vi "FlexMag - 24-03-2023.vi"() -> ()   [LabVIEW 2018] (continued)
                                }
                                frame True {
                                n21945 = Wait (ms)(milliseconds to wait=u32 100) -> ()  [unwired: 1 out]
                                "coating ch4 led 6" <- TRUE ("coating ch2 led 1")
                                }
                                }
                                }
                                frame True {
                                }
                                }
                                }
                                }
                                }
                                frame #7 {
                                # "baratron bv open"
                                n21946 = stacked-sequence {
                                frame #0 {
                                n21947 = local read "abort ch4"() -> (w25919:bool)
                                n21948 = case shown="False" w25919 {
                                frame False {
                                n21949 = local read "coating start"() -> (w25920:bool)
                                n21950 = case shown="True" w25920 {
                                frame False {
                                }
                                frame True {
                                n21951 = while {
                                i -> [w25923]
                                stop <- w25925 stop-if-true
                                n21952 = Greater Or Equal?(x=w25923, y=100) -> (x >= y?=w25924:bool)
                                n21953 = case shown="True" w25924 {
                                frame False {
                                }
                                frame True {
                                n21954 = local write "Warning Message"("Automatic Coating Process is canceled !\nCH4 Baratron Gauge Block Valve couldn't be opned.." ("Warning Message")) -> ()
                                n21955 = local write "coating error"(TRUE ("coating error")) -> ()
                                }
                                }
                                n21956 = local read "CH4_BG_BV_DI"() -> (w25929:bool)
                                n21957 = case shown="False" w25929 {
                                tunnel: [FALSE ("CH2_WFC_DO") TRUE ("CH2_WFC_DO")] -> w25928
                                frame False {
                                n21958 = Wait Until Next ms Multiple(millisecond multiple=u32 200) -> ()  [unwired: 1 out]
                                n21959 = local write "CH4_BG_BV_DO"(TRUE ("coating error")) -> ()
                                }
                                frame True {
                                }
                                }
                                n21960 = local read "coating start"() -> (w25927:bool)
                                n21961 = local read "abort ch4"() -> (w25921:bool)
                                n21962 = Not(x=w25927) -> (.not. x?=w25926:bool)
                                n21963 = Compound Arithmetic op=OR(w25928, w25926, w25921) -> (w25925:bool)
                                }
                                }
                                }
                                }
                                frame True {
                                }
                                }
                                }
                                frame #1 {
                                n21964 = local read "abort ch4"() -> (w25936:bool)
                                n21965 = case shown="False" w25936 {
                                frame False {
                                n21966 = local read "coating start"() -> (w25937:bool)
                                n21967 = case shown="True" w25937 {
                                frame False {
                                }
                                frame True {
                                n21968 = Wait (ms)(milliseconds to wait=u32 100) -> ()  [unwired: 1 out]
                                "coating ch4 led 7" <- TRUE ("coating ch2 led 1")
                                }
                                }
                                }
                                frame True {
                                }
                                }
                                }
                                }
                                }
                                frame #8 {
                                # "ar sov open"
                                n21969 = stacked-sequence {
                                frame #0 {
                                n21970 = local read "abort ch4"() -> (w25940:bool)
                                n21971 = case shown="False" w25940 {
                                frame False {
                                n21972 = local read "coating start"() -> (w25941:bool)
                                n21973 = case shown="True" w25941 {
                                frame False {
                                }
                                frame True {
                                n21974 = while {
                                i -> [w25944]
                                stop <- w25946 stop-if-true
                                n21975 = Greater Or Equal?(x=w25944, y=100) -> (x >= y?=w25945:bool)
                                n21976 = case shown="True" w25945 {
                                frame False {
                                }
                                frame True {
                                n21977 = local write "Warning Message"("Automatic Coating Process is canceled !\nCH4 SoV Ar couldn't be opened.." ("Warning Message")) -> ()
                                n21978 = local write "coating error"(TRUE ("coating error")) -> ()
                                }
                                }
                                n21979 = local read "CH4_SoV_Ar_DI"() -> (w25950:bool)
                                n21980 = case shown="False" w25950 {
                                tunnel: [FALSE ("CH2_WFC_DO") TRUE ("CH2_WFC_DO")] -> w25949
                                frame False {
                                n21981 = Wait Until Next ms Multiple(millisecond multiple=u32 200) -> ()  [unwired: 1 out]
                                n21982 = local write "CH4_SoV_Ar_DO"(TRUE ("coating error")) -> ()
                                }
                                frame True {
                                }
                                }
                                n21983 = local read "coating start"() -> (w25948:bool)
                                n21984 = local read "abort ch4"() -> (w25942:bool)
                                n21985 = Not(x=w25948) -> (.not. x?=w25947:bool)
                                n21986 = Compound Arithmetic op=OR(w25949, w25947, w25942) -> (w25946:bool)
                                }
                                }
                                }
                                }
                                frame True {
                                }
                                }
                                }
                                frame #1 {
                                n21987 = local read "abort ch4"() -> (w25957:bool)
                                n21988 = case shown="False" w25957 {
                                frame False {
                                n21989 = local read "coating start"() -> (w25958:bool)
                                n21990 = case shown="True" w25958 {
                                frame False {
                                }
                                frame True {
                                n21991 = Wait (ms)(milliseconds to wait=u32 100) -> ()  [unwired: 1 out]
                                "coating ch4 led 8" <- TRUE ("coating ch2 led 1")
                                }
                                }
                                }
                                frame True {
                                }
                                }
                                }
                                }
                                }
                                frame #9 {
                                # "mfc set"
                                n21992 = stacked-sequence {
                                frame #0 {
                                n21993 = local read "abort ch4"() -> (w25961:bool)
                                n21994 = case shown="False" w25961 {
                                frame False {
                                n21995 = local read "coating start"() -> (w25962:bool)
                                n21996 = case shown="True" w25962 {
                                frame False {
                                }
                                frame True {
                                n21997 = flat-sequence {
                                frame #0 {
                                n21998 = local read "R Ar set sccm"() -> (w25964:dbl)
                                n21999 = local write "ch4 argon mfc set"(w25964) -> ()
                                n22000 = Wait (ms)(milliseconds to wait=u32 300) -> ()  [unwired: 1 out]
                                }
                                frame #1 {
                                n22001 = local write "ch4 ar set auto"(TRUE ("ch2 ar set auto")) -> ()
                                }
                                }
                                }
                                }
                                }
                                frame True {
                                }
                                }
                                }
                                frame #1 {
                                n22002 = local read "abort ch4"() -> (w25966:bool)
                                n22003 = case shown="False" w25966 {
                                frame False {
                                n22004 = local read "coating start"() -> (w25967:bool)
                                n22005 = case shown="True" w25967 {
                                frame False {
                                }
                                frame True {
                                n22006 = while {
                                i -> [w25977]
                                stop <- w25979 stop-if-true
                                n22007 = local read "R Ar set sccm"() -> (w25973:dbl)
                                n22008 = Greater Or Equal?(x=w25977, y=50) -> (x >= y?=w25978:bool)
                                n22009 = case shown="True" w25978 {
                                frame False {
                                }
                                frame True {
                                n22010 = local write "Warning Message"("Automatic Coating Process is canceled !\nCH4  MFC Ar flow problem..." ("Warning Message")) -> ()
                                n22011 = local write "coating error"(TRUE ("coating error")) -> ()
                                }
                                }
                                n22012 = local read "ch4 argon mfc actual"() -> (w25974:dbl)
                                n22013 = Add(x=w25973, y=5.0) -> (x+y=w25970:dbl)
                                n22014 = Subtract(x=w25973, y=5.0) -> (x-y=w25969:dbl)
                                n22015 = In Range and Coerce(upper limit=w25970, x=w25974, lower limit=w25969) -> (In Range?=w25968:bool)  [unwired: 1 out]
                                n22016 = case shown="False" w25968 {
                                tunnel: [FALSE ("CH2_WFC_DO") TRUE ("CH2_WFC_DO")] -> w25982
                                frame False {
                                n22017 = Wait Until Next ms Multiple(millisecond multiple=u32 1000) -> ()  [unwired: 1 out]
                                n22018 = local write "ch4 ar set auto"(TRUE ("coating error")) -> ()
                                }
                                frame True {
                                }
                                }
                                n22019 = local read "coating start"() -> (w25981:bool)
                                n22020 = local read "abort ch4"() -> (w25975:bool)
                                n22021 = Not(x=w25981) -> (.not. x?=w25980:bool)
                                n22022 = Compound Arithmetic op=OR(w25982, w25980, w25975) -> (w25979:bool)
                                }
                                }
                                }
                                }
                                frame True {
                                }
                                }
                                }
                                frame #2 {
                                n22023 = local read "abort ch4"() -> (w25989:bool)
                                n22024 = case shown="False" w25989 {
                                frame False {
                                n22025 = local read "coating start"() -> (w25990:bool)
                                n22026 = case shown="True" w25990 {
                                frame False {
                                }
                                frame True {
                                n22027 = Wait (ms)(milliseconds to wait=u32 100) -> ()  [unwired: 1 out]
                                "coating ch4 led 9" <- TRUE ("coating ch2 led 1")
                                }
                                }
                                }
                                frame True {
                                }
                                }
                                }
                                }
                                }
                                frame #10 {
                                # "baratron pressure set"
                                n22028 = stacked-sequence {
                                frame #0 {
                                n22029 = local read "abort ch4"() -> (w25993:bool)
                                n22030 = case shown="False" w25993 {
                                frame False {
                                n22031 = local read "coating start"() -> (w25994:bool)
                                n22032 = case shown="True" w25994 {
                                frame False {
                                }
                                frame True {
                                n22033 = flat-sequence {
                                frame #0 {
                                n22034 = local read "R Pressure set mbar"() -> (w25995:dbl)
                                n22035 = Wait (ms)(milliseconds to wait=u32 300) -> ()  [unwired: 1 out]
                                n22036 = local write "pcgv4 set pressure value mbar"(w25995) -> ()
                                }
                                frame #1 {
                                n22037 = local write "pcgv4 auto set pressure"(TRUE ("ch2 ar set auto")) -> ()
                                }
                                }
                                }
                                }
                                }
                                frame True {
                                }
                                }
                                }
                                frame #1 {
                                n22038 = local read "abort ch4"() -> (w25998:bool)
                                n22039 = case shown="False" w25998 {
                                frame False {
                                n22040 = local read "coating start"() -> (w25999:bool)
                                n22041 = case shown="True" w25999 {
                                frame False {
                                }
                                frame True {
                                n22042 = while {
                                i -> [w26009]
                                stop <- w26011 stop-if-true
                                n22043 = local read "R Pressure set mbar"() -> (w26005:dbl)
                                n22044 = Greater Or Equal?(x=w26009, y=50) -> (x >= y?=w26010:bool)
                                n22045 = case shown="True" w26010 {
                                frame False {
                                }
                                frame True {
                                n22046 = local write "Warning Message"("Automatic Coating Process is canceled !\nCH4 Baratron Pressure Set problem..." ("Warning Message")) -> ()
                                n22047 = local write "coating error"(TRUE ("coating error")) -> ()
                                }
                                }
                                n22048 = local read "Ch4_baratron_pressure_mbar"() -> (w26006:dbl)
                                n22049 = Add(x=w26005, y=0.003) -> (x+y=w26002:dbl)
                                n22050 = Subtract(x=w26005, y=0.003) -> (x-y=w26001:dbl)
                                n22051 = In Range and Coerce(upper limit=w26002, x=w26006, lower limit=w26001) -> (In Range?=w26000:bool)  [unwired: 1 out]
                                n22052 = case shown="False" w26000 {
                                tunnel: [FALSE ("CH2_WFC_DO") TRUE ("CH2_WFC_DO")] -> w26014
                                frame False {
                                n22053 = Wait Until Next ms Multiple(millisecond multiple=u32 1000) -> ()  [unwired: 1 out]
                                n22054 = local write "pcgv4 auto set pressure"(TRUE ("coating error")) -> ()
                                }
                                frame True {
                                }
                                }
                                n22055 = local read "coating start"() -> (w26013:bool)
                                n22056 = local read "abort ch4"() -> (w26007:bool)
                                n22057 = Not(x=w26013) -> (.not. x?=w26012:bool)
                                n22058 = Compound Arithmetic op=OR(w26014, w26012, w26007) -> (w26011:bool)
                                }
                                }
                                }
                                }
                                frame True {
                                }
                                }
                                }
                                frame #2 {
                                n22059 = local read "abort ch4"() -> (w26021:bool)
                                n22060 = case shown="False" w26021 {
                                frame False {
                                n22061 = local read "coating start"() -> (w26022:bool)
                                n22062 = case shown="True" w26022 {
                                frame False {
                                }
                                frame True {
                                n22063 = Wait (ms)(milliseconds to wait=u32 100) -> ()  [unwired: 1 out]
                                "coating ch4 led 10" <- TRUE ("coating ch2 led 1")
                                }
                                }
                                }
                                frame True {
                                }
                                }
                                }
                                }
                                }
                                frame #11 {
                                # "power set"
                                n22064 = stacked-sequence {
                                frame #0 {
                                n22065 = local read "abort ch4"() -> (w26025:bool)
                                n22066 = case shown="False" w26025 {
                                frame False {
                                n22067 = local read "coating start"() -> (w26026:bool)
                                n22068 = case shown="True" w26026 {
                                frame False {
                                }
                                frame True {
                                n22069 = flat-sequence {
                                frame #0 {
                                n22070 = local write "RF_auto_off"(TRUE ("Dc_auto_off")) -> ()
                                }
                                frame #1 {
                                n22071 = local write "RF_forward_power_1"(i16 200 ("RF_forward_power_1")) -> ()
                                n22072 = Wait (ms)(milliseconds to wait=u32 1000) -> ()  [unwired: 1 out]
                                }
                                frame #2 {
                                n22073 = local write "RF_auto_set"(TRUE ("Dc_auto_set")) -> ()
                                }
                                }
                                }
                                }
                                }
                                frame True {
                                }
                                }
                                }
                                frame #1 {
                                n22074 = local read "abort ch4"() -> (w26031:bool)
                                n22075 = case shown="False" w26031 {
                                frame False {
                                n22076 = local read "coating start"() -> (w26032:bool)
                                n22077 = case shown="True" w26032 {
                                frame False {
                                }
                                frame True {
                                n22078 = flat-sequence {
                                frame #0 {
                                n22079 = local read "R web thickness"() -> (w26047:dbl)
                                n22080 = local read "R core diameter"() -> (w26048:dbl)
                                n22081 = local read "R tension value"() -> (w26046:dbl)
                                n22082 = local read "R web speed"() -> (w26033:dbl)
                                n22083 = local read "R rf step length 10"() -> (w26036:dbl)
                                n22084 = local read "R rf step length 1"() -> (w26045:dbl)
                                n22085 = local read "R rf step length 2"() -> (w26044:dbl)
                                n22086 = local read "R rf step length 3"() -> (w26043:dbl)
                                n22087 = local read "R rf step length 4"() -> (w26042:dbl)
                                n22088 = local read "R rf step length 5"() -> (w26041:dbl)
                                n22089 = local read "R rf step length 6"() -> (w26040:dbl)
                                n22090 = local read "R rf step length 7"() -> (w26039:dbl)
                                n22091 = local read "R rf step length 8"() -> (w26038:dbl)
                                n22092 = local read "R rf step length 9"() -> (w26037:dbl)
                                n22093 = local write "web speed"(w26033) -> ()
                                n22094 = local write "setpoint"(w26033) -> ()
                                n22095 = local write "initial right diameter"(w26048) -> ()
                                n22096 = local write "web thickness"(w26047) -> ()
                                n22097 = local write "tension value"(w26046) -> ()
                                n22098 = Compound Arithmetic op=ADD(w26045, w26044, w26043, w26042, w26041, w26040, w26039, w26038, w26037, w26036) -> (w26035:dbl)
                                n22099 = local write "target interval"(w26035) -> ()
                                n22100 = Wait (ms)(milliseconds to wait=u32 500) -> ()  [unwired: 1 out]
                                }
                                frame #1 {
                                n22101 = Wait (ms)(milliseconds to wait=u32 500) -> ()  [unwired: 1 out]
                                }
                                frame #2 {
                                n22102 = local write "calculate"(TRUE ("calculate")) -> ()
                                }
                                }
                                }
                                }
                                }
                                frame True {
                                }
                                }
                                }
                                frame #2 {
                                n22103 = local read "abort ch4"() -> (w26051:bool)
                                n22104 = case shown="False" w26051 {
                                frame False {
                                n22105 = local read "coating start"() -> (w26052:bool)
                                n22106 = case shown="True" w26052 {
                                frame False {
                                }
                                frame True {
                                n22107 = flat-sequence {
                                frame #0 {
                                n22108 = while {
                                i -> [w26057]
                                stop <- w26053 stop-if-true
                                n22109 = local read "coating start"() -> (w26061:bool)
                                n22110 = local read "calculate"() -> (w26062:bool)
                                n22111 = local read "abort ch4"() -> (w26060:bool)
                                n22112 = Greater Or Equal?(x=w26057, y=60) -> (x >= y?=w26054:bool)
                                n22113 = Not(x=w26062) -> (.not. x?=w26058:bool)
                                n22114 = Not(x=w26061) -> (.not. x?=w26059:bool)
                                n22115 = Wait Until Next ms Multiple(millisecond multiple=u32 1000) -> ()  [unwired: 1 out]
                                n22116 = Compound Arithmetic op=OR(w26054, w26058, w26059, w26060) -> (w26053:bool)
                                }
                                }
                                frame #1 {
                                n22117 = local read "R RF number steps"() -> (w26064:dbl)
                                n22118 = Wait (ms)(milliseconds to wait=u32 1000) -> ()  [unwired: 1 out]
                                n22119 = local write "current step"(0.0 ("step count")) -> ()
                                n22120 = local write "step count"(w26064) -> ()
                                }
                                }
                                }
                                }
                                }
                                frame True {
                                }
                                }
                                }
                                frame #3 {
                                n22121 = local read "abort ch4"() -> (w26066:bool)
                                n22122 = case shown="False" w26066 {
                                frame False {
                                n22123 = local read "coating start"() -> (w26067:bool)
                                n22124 = case shown="True" w26067 {
                                frame False {
                                }
                                frame True {
                                n22125 = flat-sequence {
                                frame #0 {
                                n22126 = local read "dep. for?"() -> (w26068:bool)
                                n22127 = case shown="False" w26068 {
                                frame False {
                                n22128 = local write "back roll"(TRUE ("back roll")) -> ()
                                }
                                frame True {
                                n22129 = local write "forward roll"(TRUE ("forward roll")) -> ()
                                }
                                }
                                }
                                frame #1 {
                                n22130 = Wait (ms)(milliseconds to wait=u32 1000) -> ()  [unwired: 1 out]
                                }
                                frame #2 {
                                n22131 = while {
                                i -> [w26077]
                                stop <- w26074 stop-if-true
                                n22132 = local read "CH4_Motor DO"() -> (w26073:bool)
                                n22133 = local read "coating start"() -> (w26080:bool)
                                n22134 = Wait Until Next ms Multiple(millisecond multiple=u32 1000) -> ()  [unwired: 1 out]
                                n22135 = local read "abort ch4"() -> (w26079:bool)
                                n22136 = Greater Or Equal?(x=w26077, y=60) -> (x >= y?=w26072:bool)
                                n22137 = Not(x=w26080) -> (.not. x?=w26078:bool)
                                n22138 = local write "RF_auto_on"(w26073) -> ()
                                n22139 = local write "coating error"(w26072) -> ()
                                n22140 = Compound Arithmetic op=OR(w26073, w26078, w26079, w26072) -> (w26074:bool)
                                }
                                }
                                frame #3 {
                                n22141 = Wait (ms)(milliseconds to wait=u32 500) -> ()  [unwired: 1 out]
                                }
                                }
                                }
                                }
                                }
                                frame True {
                                }
                                }
                                }
                                frame #4 {
                                n22142 = local read "abort ch4"() -> (w26082:bool)
                                n22143 = case shown="False" w26082 {
                                frame False {
                                n22144 = local read "coating start"() -> (w26083:bool)
                                n22145 = case shown="True" w26083 {
                                frame False {
                                }
                                frame True {
                                }
                                }
                                }
                                frame True {
                                }
                                }
                                }
                                frame #5 {
                                n22146 = local read "abort ch4"() -> (w26084:bool)
                                n22147 = case shown="False" w26084 {
                                frame False {
                                n22148 = local read "coating start"() -> (w26085:bool)
                                n22149 = case shown="True" w26085 {
                                frame False {
                                }
                                frame True {
                                n22150 = Wait (ms)(milliseconds to wait=u32 100) -> ()  [unwired: 1 out]
                                "coating ch4 led 11" <- TRUE ("coating ch2 led 1")
                                }
                                }
                                }
                                frame True {
                                }
                                }
                                }
                                }
                                }
                                frame #12 {
                                # "power steps"
                                n22151 = disable-structure shown="Enabled" {
                                frame Disabled {
                                n22152 = stacked-sequence {
                                frame #0 {
                                n22153 = local read "abort ch2"() -> (w26088:bool)
                                n22154 = case shown="False" w26088 {
                                frame False {
                                n22155 = local read "coating start"() -> (w26089:bool)
                                n22156 = case shown="True" w26089 {
                                frame False {
                                }
                                frame True {
                                n22157 = local read "R dc step length 1"() -> (w26092:dbl)
                                n22158 = Greater?(x=w26092, y=0.0) -> (0:w26091:bool)
                                n22159 = case shown="True" w26091 {
                                frame False {
                                }
                                frame True {
                                n22160 = flat-sequence {
                                frame #0 {
                                n22161 = local read "R dc step length 1"() -> (w26099:dbl)
                                n22162 = local read "R dc step power 1"() -> (w26094:dbl)
                                n22163 = local read "R web speed"() -> (w26098:dbl)
                                n22164 = Divide(x=w26099, y=w26098) -> (x/y=w26097:dbl)
                                n22165 = local write "Set DC Power ch2"(w26094) -> ()
                                n22166 = Multiply(x=w26097, y=60) -> (x*y=w26095:dbl)
                                n22167 = Wait (ms)(milliseconds to wait=u32 100) -> ()  [unwired: 1 out]
                                n22168 = local write "time counting"(w26095) -> ()
                                }
                                frame #1 {
                                n22169 = local write "Dc_auto_set"(TRUE ("Dc_auto_set")) -> ()
                                }
                                frame #2 {
                                n22170 = while {
                                stop <- w26102 stop-if-true
                                n22171 = local read "time counting"() -> (w26108:dbl)
                                n22172 = Wait Until Next ms Multiple(millisecond multiple=u32 1000) -> ()  [unwired: 1 out]
                                n22173 = local read "coating start"() -> (w26106:bool)
                                n22174 = local read "abort ch2"() -> (w26104:bool)
                                n22175 = Decrement(x=w26108) -> (x-1=w26107:dbl)
                                n22176 = local write "time counting"(w26107) -> ()
                                n22177 = Not(x=w26106) -> (.not. x?=w26105:bool)
                                n22178 = Less Or Equal To 0?(x=w26107) -> (x <= 0?=w26103:bool)
                                n22179 = Compound Arithmetic op=OR(w26103, w26105, w26104) -> (w26102:bool)
                                }
                                }
                                }
                                }
                                }
                                }
                                }
                                }
                                frame True {
                                }
                                }
                                }
                                frame #1 {
                                n22180 = local read "abort ch2"() -> (w26109:bool)
                                n22181 = case shown="False" w26109 {
                                frame False {
                                n22182 = local read "coating start"() -> (w26110:bool)
                                n22183 = case shown="True" w26110 {
                                frame False {
                                }
                                frame True {
                                n22184 = local read "R dc step length 2"() -> (w26113:dbl)
                                n22185 = Greater?(x=w26113, y=0.0) -> (0:w26112:bool)
                                n22186 = case shown="True" w26112 {
                                frame False {
                                }
                                frame True {
                                n22187 = flat-sequence {
                                frame #0 {
                                n22188 = local read "R dc step length 2"() -> (w26120:dbl)
                                n22189 = local read "R dc step power 2"() -> (w26115:dbl)
                                n22190 = local read "R web speed"() -> (w26119:dbl)
                                n22191 = Divide(x=w26120, y=w26119) -> (x/y=w26118:dbl)
                                n22192 = local write "Set DC Power ch2"(w26115) -> ()
                                n22193 = Multiply(x=w26118, y=60) -> (x*y=w26116:dbl)
                                n22194 = Wait (ms)(milliseconds to wait=u32 100) -> ()  [unwired: 1 out]
                                n22195 = local write "time counting"(w26116) -> ()
                                }
                                frame #1 {
                                n22196 = local write "Dc_auto_set"(TRUE ("Dc_auto_set")) -> ()
                                }
                                frame #2 {
                                n22197 = while {
                                stop <- w26123 stop-if-true
                                n22198 = local read "time counting"() -> (w26129:dbl)
                                n22199 = local read "coating start"() -> (w26127:bool)
                                n22200 = local read "abort ch2"() -> (w26125:bool)
                                n22201 = Wait Until Next ms Multiple(millisecond multiple=u32 1000) -> ()  [unwired: 1 out]
                                n22202 = Decrement(x=w26129) -> (x-1=w26128:dbl)
                                n22203 = local write "time counting"(w26128) -> ()
                                n22204 = Not(x=w26127) -> (.not. x?=w26126:bool)
                                n22205 = Less Or Equal To 0?(x=w26128) -> (x <= 0?=w26124:bool)
                                n22206 = Compound Arithmetic op=OR(w26124, w26126, w26125) -> (w26123:bool)
                                }
                                }
                                }
                                }
                                }
                                }
                                }
                                }
                                frame True {
                                }
                                }
                                }
                                frame #2 {
                                n22207 = local read "abort ch2"() -> (w26130:bool)
                                n22208 = case shown="False" w26130 {
                                frame False {
                                n22209 = local read "coating start"() -> (w26131:bool)
                                n22210 = case shown="True" w26131 {
                                frame False {
                                }
                                frame True {
                                n22211 = local read "R dc step length 3"() -> (w26134:dbl)
                                n22212 = Greater?(x=w26134, y=0.0) -> (0:w26133:bool)
                                n22213 = case shown="True" w26133 {
                                frame False {
                                }
                                frame True {
                                n22214 = flat-sequence {
                                frame #0 {
                                n22215 = local read "R dc step length 3"() -> (w26141:dbl)
                                n22216 = local read "R dc step power 3"() -> (w26136:dbl)
                                n22217 = local read "R web speed"() -> (w26140:dbl)
                                n22218 = Divide(x=w26141, y=w26140) -> (x/y=w26139:dbl)
                                n22219 = local write "Set DC Power ch2"(w26136) -> ()
                                n22220 = Multiply(x=w26139, y=60) -> (x*y=w26137:dbl)
                                n22221 = Wait (ms)(milliseconds to wait=u32 100) -> ()  [unwired: 1 out]
                                n22222 = local write "time counting"(w26137) -> ()
                                }
                                frame #1 {
                                n22223 = local write "Dc_auto_set"(TRUE ("Dc_auto_set")) -> ()
                                }
                                frame #2 {
                                n22224 = while {
                                stop <- w26144 stop-if-true
                                n22225 = local read "time counting"() -> (w26150:dbl)
                                n22226 = local read "coating start"() -> (w26148:bool)
                                n22227 = Wait Until Next ms Multiple(millisecond multiple=u32 1000) -> ()  [unwired: 1 out]
                                n22228 = local read "abort ch2"() -> (w26146:bool)
                                n22229 = Decrement(x=w26150) -> (x-1=w26149:dbl)
                                n22230 = local write "time counting"(w26149) -> ()
                                n22231 = Not(x=w26148) -> (.not. x?=w26147:bool)
                                n22232 = Less Or Equal To 0?(x=w26149) -> (x <= 0?=w26145:bool)
                                n22233 = Compound Arithmetic op=OR(w26145, w26147, w26146) -> (w26144:bool)
                                }
                                }
                                }
                                }
                                }
                                }
                                }
                                }
                                frame True {
                                }
                                }
                                }
                                frame #3 {
                                n22234 = local read "abort ch2"() -> (w26151:bool)
                                n22235 = case shown="False" w26151 {
                                frame False {
                                n22236 = local read "coating start"() -> (w26152:bool)
                                n22237 = case shown="True" w26152 {
                                frame False {
                                }
                                frame True {
                                n22238 = local read "R dc step length 4"() -> (w26155:dbl)
                                n22239 = Greater?(x=w26155, y=0.0) -> (0:w26154:bool)
                                n22240 = case shown="True" w26154 {
                                frame False {
                                }
                                frame True {
                                n22241 = flat-sequence {
                                frame #0 {
                                n22242 = local read "R dc step length 4"() -> (w26162:dbl)
                                n22243 = local read "R dc step power 4"() -> (w26157:dbl)
                                n22244 = local read "R web speed"() -> (w26161:dbl)
                                n22245 = Divide(x=w26162, y=w26161) -> (x/y=w26160:dbl)
                                n22246 = local write "Set DC Power ch2"(w26157) -> ()
                                n22247 = Wait (ms)(milliseconds to wait=u32 100) -> ()  [unwired: 1 out]
                                n22248 = Multiply(x=w26160, y=60) -> (x*y=w26158:dbl)
                                n22249 = local write "time counting"(w26158) -> ()
                                }
                                frame #1 {
                                n22250 = local write "Dc_auto_set"(TRUE ("Dc_auto_set")) -> ()
                                }
                                frame #2 {
                                n22251 = while {
                                stop <- w26165 stop-if-true
                                n22252 = local read "time counting"() -> (w26171:dbl)
                                n22253 = local read "coating start"() -> (w26169:bool)
                                n22254 = local read "abort ch2"() -> (w26167:bool)
                                n22255 = Wait Until Next ms Multiple(millisecond multiple=u32 1000) -> ()  [unwired: 1 out]
                                n22256 = Decrement(x=w26171) -> (x-1=w26170:dbl)
                                n22257 = local write "time counting"(w26170) -> ()
                                n22258 = Not(x=w26169) -> (.not. x?=w26168:bool)
                                n22259 = Less Or Equal To 0?(x=w26170) -> (x <= 0?=w26166:bool)
                                n22260 = Compound Arithmetic op=OR(w26166, w26168, w26167) -> (w26165:bool)
                                }
                                }
                                }
                                }
                                }
                                }
                                }
                                }
                                frame True {
                                }
                                }
                                }
                                frame #4 {
                                n22261 = local read "abort ch2"() -> (w26172:bool)
                                n22262 = case shown="False" w26172 {
                                frame False {
                                n22263 = local read "coating start"() -> (w26173:bool)
                                n22264 = case shown="True" w26173 {
                                frame False {
                                }
                                frame True {
                                n22265 = local read "R dc step length 5"() -> (w26176:dbl)
                                n22266 = Greater?(x=w26176, y=0.0) -> (0:w26175:bool)
                                n22267 = case shown="True" w26175 {
                                frame False {
                                }
                                frame True {
                                n22268 = flat-sequence {
                                frame #0 {
                                n22269 = local read "R dc step length 5"() -> (w26183:dbl)
                                n22270 = local read "R dc step power 5"() -> (w26178:dbl)
                                n22271 = local read "R web speed"() -> (w26182:dbl)
                                n22272 = Divide(x=w26183, y=w26182) -> (x/y=w26181:dbl)
                                n22273 = Wait (ms)(milliseconds to wait=u32 100) -> ()  [unwired: 1 out]
                                n22274 = local write "Set DC Power ch2"(w26178) -> ()
                                n22275 = Multiply(x=w26181, y=60) -> (x*y=w26179:dbl)
                                n22276 = local write "time counting"(w26179) -> ()
                                }
                                frame #1 {
                                n22277 = local write "Dc_auto_set"(TRUE ("Dc_auto_set")) -> ()
                                }
                                frame #2 {
                                n22278 = while {
                                stop <- w26186 stop-if-true
                                n22279 = local read "time counting"() -> (w26192:dbl)
                                n22280 = local read "coating start"() -> (w26190:bool)
                                n22281 = Wait Until Next ms Multiple(millisecond multiple=u32 1000) -> ()  [unwired: 1 out]
                                n22282 = local read "abort ch2"() -> (w26188:bool)
                                n22283 = Decrement(x=w26192) -> (x-1=w26191:dbl)
                                n22284 = local write "time counting"(w26191) -> ()
                                n22285 = Not(x=w26190) -> (.not. x?=w26189:bool)
                                n22286 = Less Or Equal To 0?(x=w26191) -> (x <= 0?=w26187:bool)
                                n22287 = Compound Arithmetic op=OR(w26187, w26189, w26188) -> (w26186:bool)
                                }
                                }
                                }
                                }
                                }
                                }
                                }
                                }
                                frame True {
                                }
                                }
                                }
                                frame #5 {
                                n22288 = local read "abort ch2"() -> (w26193:bool)
                                n22289 = case shown="False" w26193 {
                                frame False {
                                n22290 = local read "coating start"() -> (w26194:bool)
                                n22291 = case shown="True" w26194 {
                                frame False {
                                }
                                frame True {
                                n22292 = local read "R dc step length 6"() -> (w26197:dbl)
                                n22293 = Greater?(x=w26197, y=0.0) -> (0:w26196:bool)
                                n22294 = case shown="True" w26196 {
                                frame False {
                                }
                                frame True {
                                n22295 = flat-sequence {
                                frame #0 {
                                n22296 = local read "R dc step length 6"() -> (w26204:dbl)
                                n22297 = local read "R dc step power 6"() -> (w26199:dbl)
                                n22298 = local read "R web speed"() -> (w26203:dbl)
                                n22299 = Wait (ms)(milliseconds to wait=u32 100) -> ()  [unwired: 1 out]
                                n22300 = Divide(x=w26204, y=w26203) -> (x/y=w26202:dbl)
                                n22301 = local write "Set DC Power ch2"(w26199) -> ()
                                n22302 = Multiply(x=w26202, y=60) -> (x*y=w26200:dbl)
                                n22303 = local write "time counting"(w26200) -> ()
                                }
                                frame #1 {
                                n22304 = local write "Dc_auto_set"(TRUE ("Dc_auto_set")) -> ()
                                }
                                frame #2 {
                                n22305 = while {
                                stop <- w26207 stop-if-true
                                n22306 = local read "time counting"() -> (w26213:dbl)
                                n22307 = local read "coating start"() -> (w26211:bool)
                                n22308 = local read "abort ch2"() -> (w26209:bool)
                                n22309 = Wait Until Next ms Multiple(millisecond multiple=u32 1000) -> ()  [unwired: 1 out]
                                n22310 = Decrement(x=w26213) -> (x-1=w26212:dbl)
                                n22311 = local write "time counting"(w26212) -> ()
                                n22312 = Not(x=w26211) -> (.not. x?=w26210:bool)
                                n22313 = Less Or Equal To 0?(x=w26212) -> (x <= 0?=w26208:bool)
                                n22314 = Compound Arithmetic op=OR(w26208, w26210, w26209) -> (w26207:bool)
                                }
                                }
                                }
                                }
                                }
                                }
                                }
                                }
                                frame True {
                                }
                                }
                                }
                                frame #6 {
                                n22315 = local read "abort ch2"() -> (w26214:bool)
                                n22316 = case shown="False" w26214 {
                                frame False {
                                n22317 = local read "coating start"() -> (w26215:bool)
                                n22318 = case shown="True" w26215 {
                                frame False {
                                }
                                frame True {
                                n22319 = local read "R dc step length 7"() -> (w26218:dbl)
                                n22320 = Greater?(x=w26218, y=0.0) -> (0:w26217:bool)
                                n22321 = case shown="True" w26217 {
                                frame False {
                                }
                                frame True {
                                n22322 = flat-sequence {
                                frame #0 {
                                n22323 = local read "R dc step length 7"() -> (w26225:dbl)
                                n22324 = local read "R dc step power 7"() -> (w26220:dbl)
                                n22325 = local read "R web speed"() -> (w26224:dbl)
                                n22326 = Divide(x=w26225, y=w26224) -> (x/y=w26223:dbl)
                                n22327 = Wait (ms)(milliseconds to wait=u32 100) -> ()  [unwired: 1 out]
                                n22328 = local write "Set DC Power ch2"(w26220) -> ()
                                n22329 = Multiply(x=w26223, y=60) -> (x*y=w26221:dbl)
                                n22330 = local write "time counting"(w26221) -> ()
                                }
                                frame #1 {
                                n22331 = local write "Dc_auto_set"(TRUE ("Dc_auto_set")) -> ()
                                }
                                frame #2 {
                                n22332 = while {
                                stop <- w26228 stop-if-true
                                n22333 = local read "time counting"() -> (w26234:dbl)
                                n22334 = local read "coating start"() -> (w26232:bool)
                                n22335 = local read "abort ch2"() -> (w26230:bool)
                                n22336 = Wait Until Next ms Multiple(millisecond multiple=u32 1000) -> ()  [unwired: 1 out]
                                n22337 = Decrement(x=w26234) -> (x-1=w26233:dbl)
                                n22338 = local write "time counting"(w26233) -> ()
                                n22339 = Not(x=w26232) -> (.not. x?=w26231:bool)
                                n22340 = Less Or Equal To 0?(x=w26233) -> (x <= 0?=w26229:bool)
                                n22341 = Compound Arithmetic op=OR(w26229, w26231, w26230) -> (w26228:bool)
                                }
                                }
                                }
                                }
                                }
                                }
                                }
                                }
                                frame True {
                                }
                                }
                                }
                                frame #7 {
                                n22342 = local read "abort ch2"() -> (w26235:bool)
                                n22343 = case shown="False" w26235 {
                                frame False {
                                n22344 = local read "coating start"() -> (w26236:bool)
                                n22345 = case shown="True" w26236 {
                                frame False {
                                }
                                frame True {
                                n22346 = local read "R dc step length 8"() -> (w26239:dbl)
                                n22347 = Greater?(x=w26239, y=0.0) -> (0:w26238:bool)
                                n22348 = case shown="True" w26238 {
                                frame False {
                                }
                                frame True {
                                n22349 = flat-sequence {
                                frame #0 {
                                n22350 = local read "R dc step length 8"() -> (w26246:dbl)
                                n22351 = local read "R dc step power 8"() -> (w26241:dbl)
                                n22352 = local read "R web speed"() -> (w26245:dbl)
                                n22353 = Wait (ms)(milliseconds to wait=u32 100) -> ()  [unwired: 1 out]
                                n22354 = Divide(x=w26246, y=w26245) -> (x/y=w26244:dbl)
                                n22355 = local write "Set DC Power ch2"(w26241) -> ()
                                n22356 = Multiply(x=w26244, y=60) -> (x*y=w26242:dbl)
                                n22357 = local write "time counting"(w26242) -> ()
                                }
                                frame #1 {
                                n22358 = local write "Dc_auto_set"(TRUE ("Dc_auto_set")) -> ()
                                }
                                frame #2 {
                                n22359 = while {
                                stop <- w26249 stop-if-true
                                n22360 = local read "time counting"() -> (w26255:dbl)
                                n22361 = local read "coating start"() -> (w26253:bool)